vi "HFRR ADV v037.vi"() -> ()   [LabVIEW 2025] (continued)
        n1681 = VISA Close(VISA resource name=w2091, error in (no error)=w2090) -> (error out=w2093:errorcluster)
        n1682 = call <vilib>:"Clear Errors.vi"("error in (no error)"=w2093) -> ()  [unwired: 5 in, 2 out]
        n1683 = local write "Port 2a"(FALSE ("Port 2a")) -> ()
        n1684 = local read "Com Port 2"() -> (w2086:refnum<visa-resource-name>)
        "visa due" <- w2086
        n1685 = call-poly "VISA Configure Serial Port"("VISA resource name"=w2086, "timeout (10sec)"=w2097, "baud rate (9600)"=u32 250000 ("baud rate  2"), "data bits (8)"=u16 8 ("data bits  2"), "parity (0:none)"=w2096, "stop bits (10: 1 bit)"=w2098, "flow control (0:none)"=w2100) -> ("VISA resource name out"=w2101:refnum<visa-resource-name>, "error out"=w2102:errorcluster)  [unwired: 7 in]
        n1686 = flat-sequence {
          tunnel: w2101 -> [w2104]
          tunnel: w2102 -> [w2103]
          tunnel: [w2104] -> w2094
          tunnel: [w2103] -> w2087
          frame #0 {
            n1687 = Wait (ms)(milliseconds to wait=u32 50) -> ()  [unwired: 1 out]
          }
        }
        "Residual Due" <- ""
      }
    }
    "error out 9" <- w2028
    n1688 = local read "Quit"() -> (w2030:bool)
    "Error Due" <- w2035
  }
  n1689 = local write "FRICVALZ"(0.0 ("FRICVALZ")) -> ()
  n1690 = property on="RUN" class="Bool (strict)"("Visible"=TRUE) -> ()  [unwired: 2 in, 2 out]
  n1691 = while {
    tunnel: [w2119] -> _
    tunnel: [w2106] -> w54
    i -> [w2119]
    stop <- w2106 stop-if-true
    n1692 = local read "conststatus"() -> (w2110:dbl)
    n1693 = local read "Main Tab"() -> (w2108:T2)
    n1694 = local read "EDIT"() -> (w2125:bool)
    n1695 = local read "Rate"() -> (w2124:dbl)
    n1696 = case shown="True" w2125 {
      tunnel: [FALSE TRUE] -> _
      frame False {
      }
      frame True {
      }
    }
    n1697 = Equal?(x=w2108, y=T29."About" ("Main Tab")) -> (x = y?=w2117:bool)
    n1698 = Equal?(x=w2110, y=0.0) -> (x = y?=w2111:bool)
    n1699 = Divide(x=1.0, y=w2124) -> (x/y=w2120:dbl)
    "Time 2" <- w2120
    n1700 = case shown="True" w2111 {
      frame False {
      }
      frame True {
        # "C:\\WinDucom\\calibrate WO 2391.dcf"
        n1701 = local write "Lan flag"(22) -> ()
        n1702 = local write "conststatus"(10.0 ("rpm value : 2")) -> ()
        n1703 = String To Path(string="C:\\LAB-IQ\\calibrate WO 2465.dcf") -> (path=w2131:path)
        n1704 = Open/Create/Replace File "Open File"(file path (use dialog)=w2131) -> (refnum out=w2129:refnum<file>)  [unwired: 5 in, 2 out]
        n1705 = for {
          N: 23 -> [_]
          tunnel: w2129 -> [w2140]
          i -> [w2134]
          (unwired) TRUE ("line mode (F)")
          n1706 = Read from Text File "Read File"(file (use dialog)=w2140) -> (text=w2139:string)  [unwired: 3 in, 3 out]
          n1707 = Match Pattern(string=w2139, regular expression="]") -> (after substring=w2137:string)  [unwired: 1 in, 3 out]
          n1708 = String Subset(string=w2139, offset (0)=5, length (rest)=10 ("length (rest)")) -> (substring=w2132:string)
          n1709 = Fract/Exp String To Number(string=w2132) -> (number=w2133:dbl)  [unwired: 3 in, 1 out]
          n1710 = Match Pattern(string=w2137, regular expression="-") -> (before substring=w2135:string)  [unwired: 1 in, 3 out]
          n1711 = case shown="10" w2134 {
            tunnel: w2133 -> [_ _ _ _ _ _ _ _ _ _ w2147 _ _ _ _ _ _ _ _ _ _ _ _ _]
            tunnel: w2135 -> [_ _ _ _ w2143 w2144 w2145 _ _ _ _ _ _ _ _ _ _ _ _ _ w2148 w2149 w2150 _]
            frame 0 {
            }
            frame 1 {
            }
            frame 2 {
            }
            frame 3 {
            }
            frame 4 {
              n1712 = local write "Com Port 1"(w2143) -> ()
            }
            frame 5 {
              n1713 = local write "Com Port 2"(w2144) -> ()
              n1714 = local write "visa due"(w2144) -> ()
            }
            frame 6 {
              n1715 = String To Path(string=w2145) -> (path=w2146:path)
              n1716 = local write "File Path"(w2146) -> ()
              "String" <- w2145
            }
            frame 7 {
            }
            frame 8 {
            }
            frame 9 {
            }
            frame 10 {
              n1717 = local write "Language Selection"(w2147) -> ()
            }
            frame 11 {
            }
            frame 12 {
            }
            frame 13 {
            }
            frame 14 {
            }
            frame 15 {
            }
            frame 16 {
            }
            frame 17 {
            }
            frame 18 {
            }
            frame 21 {
            }
            frame 22 {
              n1718 = local write "Com Port 3"(w2148) -> ()
            }
            frame 20 {
              n1719 = local write "Camera Port :"(w2149) -> ()
            }
            frame 19 {
              n1720 = local write "C3 :"(w2150) -> ()
            }
            frame 23, Default {
            }
          }
        }
      }
    }
    n1721 = Select(t=u32 2500 ("milliseconds to wait"), s=w2117, f=u32 500 ("milliseconds to wait")) -> (s? t:f=w2115:u32)
    n1722 = Multiply(x=w2120, y=w2115) -> (x*y=w2122:dbl)
    n1723 = call "Elapsed Time2"("Time Target (s)"=w2122, "Auto Reset"=TRUE) -> ("Time has Elapsed"=w2112:bool)  [unwired: 10 in, 7 out]
    n1724 = case shown="True" w2112 {
      frame False {
      }
      frame True {
        n1725 = stacked-sequence {
          frame #0 {
            # "DATA PROCESSING"
            # "115 mV/N"
            n1726 = local read "Sample Temperature"() -> (w2153:dbl)
            n1727 = local read "RH Numeric:"() -> (→"Humidity ( %RH )":dbl)
            n1728 = local read "FRICVALZ"() -> (w2170:dbl)
            n1729 = local read "Friction"() -> (w2156:dbl)
            n1730 = call <vilib>:"Mean PtByPt.vi"("x"=w2153, "sample length"=100) -> ("mean"=w2152:dbl)  [unwired: 2 in, 1 out]
            "TEMP 2" <- w2152
            "TEMP 3" <- w2152
            n1731 = Subtract(x=w2156, y=w2170) -> (x-y=w2165:dbl)
            "FF 2" <- w2165
            "FF 4" <- w2165
            n1732 = local read "Ambient Temperature"() -> (→"AIR TEMP":dbl)
            n1733 = local read "TEMP"() -> (w2169:dbl)
            n1734 = local write "FF 3"(w2165) -> ()
            n1735 = Compound Arithmetic op=OR("FRICVALZ 4", "FRICVALZ 3", "FRICVALZ 2") -> (w2161:bool)
            n1736 = case shown="True" w2161 {
              tunnel: w2156 -> [_ w2176]
              frame False {
              }
              frame True {
                w2175 = FALSE ("FRICVALZ")
                n1737 = local write "FRICVALZ 3"(w2175) -> ()
                n1738 = local write "FRICVALZ 2"(w2175) -> ()
                n1739 = local write "FRICVALZ 4"(w2175) -> ()
                "FRICVALZ" <- w2176
              }
            }
            n1740 = Not A Number/Path/Refnum?(number/path/refnum=w2169) -> (NaN/Path/Refnum?=w2168:bool)
            n1741 = Not A Number/Path/Refnum?(number/path/refnum=w2165) -> (NaN/Path/Refnum?=w2167:bool)
            n1742 = Divide(x=w2165, y=1.96) -> (x/y=w2162:dbl)
            n1743 = Compound Arithmetic op=OR(w2168, w2167) -> (w2166:bool)
            n1744 = Not A Number/Path/Refnum?(number/path/refnum=w2162) -> (NaN/Path/Refnum?=w2163:bool)
            n1745 = case shown="True" w2166 {
              frame False {
              }
              frame True {
                n1746 = local write "TEMP"(0.0 ("TEMP")) -> ()
                n1747 = local write "FF 2"(0.0 ("FF 2")) -> ()
                n1748 = local write "reinit"(TRUE ("reinit")) -> ()
              }
            }
            n1749 = local write "TEMP"(w2152) -> ()
            n1750 = Select(t=0.0, s=w2163, f=w2162) -> (s? t:f=w2155:dbl)
            "COF 2" <- w2155
            n1751 = local write "COF 3"(w2155) -> ()
          }
        }
      }
    }
    n1752 = Wait (ms)(milliseconds to wait=u32 50) -> ()  [unwired: 1 out]
    n1753 = local read "Quit"() -> (w2106:bool)
    "Rate" <- 2500.0 ("No of Samples")
  }
  n1754 = while {
    tunnel: [w2196] -> _
    tunnel: [w2179] -> w56
    tunnel: w1 -> [_]
    i -> [w2196]
    stop <- w2179 stop-if-true
    # "C:\\LAB-IQ-NXT\\Scar View.exe"
    n1755 = local read "OK Button 16"() -> (w2186:bool)
    n1756 = local read "Main Tab"() -> (w2180:T2)
    n1757 = local read "service 3"() -> (w2181:bool)
    n1758 = local read "OPEN 6"() -> (w2183:bool)
    n1759 = local read "EDIT 2"() -> (w2185:bool)
    n1760 = flat-sequence {
      frame #0 {
        n1761 = stacked-sequence {
          frame #0 {
            n1762 = local read "EDIT"() -> (w2674:bool)
            n1763 = case shown="False" w2674 {
              tunnel: [u8 2 ("Disabled") u8 0 ("Disabled")] -> _
              frame False {
                w2676 = FALSE
                n1764 = local write "Password"("") -> ()
                n1765 = local write "x = y?"(w2676) -> ()
                n1766 = property on="Password" class="Str"("Visible"=w2676) -> ()  [unwired: 2 in, 2 out]
              }
              frame True {
                n1767 = property on="Password" class="Str"("Visible"=TRUE) -> ()  [unwired: 2 in, 2 out]
              }
            }
            "dipl pwd" <- "@143$\n" ("dipl pwd")
          }
          frame #1 {
          }
          frame #2 {
          }
          frame #3 {
          }
          frame #4 {
            n1768 = String To Byte Array(string="Password") -> (unsigned byte array=w2687:u8[])
            n1769 = Search 1D Array(1D array=w2687, element=u8 10) -> (index of element=w2685:i32)  [unwired: 1 in]
            n1770 = Index Array(array=w2687, index=w2685) -> (element=w2686:u8)
            n1771 = Equal?(x=w2686, y=10) -> (x = y?=w2682:bool)
            n1772 = case shown="True" w2682 {
              frame False {
              }
              frame True {
                # "password"
                # "password"
                n1773 = local read "Password"() -> (w2699:string)
                n1774 = String To Byte Array(string=w2699) -> (unsigned byte array=w2702:u8[])
                n1775 = String To Byte Array(string="@143$\n") -> (unsigned byte array=w2689:u8[])
                n1776 = Array Size(array=w2702) -> (size(s)=w2698:i32)
                n1777 = Array Size(array=w2689) -> (size(s)=w2694:i32)
                n1778 = for {
                  N: w2698 -> [_]
                  tunnel: w2702 -> [w2715]
                  tunnel: [w2713] -> w2703 mode=indexing
                  tunnel: w2698 -> [w2710]
                  i -> [w2711]
                  n1779 = Decrement(x=w2710) -> (x-1=w2709:i32)
                  n1780 = Index Array(array=w2715, index=w2711) -> (element=w2714:u8)
                  n1781 = Equal?(x=w2711, y=w2709) -> (x = y?=w2708:bool)
                  n1782 = Number To Decimal String(number=w2714) -> (decimal integer string=w2712:string)  [unwired: 1 in]
                  n1783 = Select(t="", s=w2708, f="\r") -> (s? t:f=w2705:string)
                  n1784 = Concatenate Strings(w2712, w2705) -> (w2713:string)
                }
                n1785 = for {
                  N: w2694 -> [_]
                  tunnel: w2689 -> [w2726]
                  tunnel: [w2724] -> w2692 mode=indexing
                  tunnel: w2694 -> [w2721]
                  i -> [w2722]
                  n1786 = Decrement(x=w2721) -> (x-1=w2720:i32)
                  n1787 = Index Array(array=w2726, index=w2722) -> (element=w2725:u8)
                  n1788 = Equal?(x=w2722, y=w2720) -> (x = y?=w2719:bool)
                  n1789 = Number To Decimal String(number=w2725) -> (decimal integer string=w2723:string)  [unwired: 1 in]
                  n1790 = Select(t="", s=w2719, f="\r") -> (s? t:f=w2716:string)
                  n1791 = Concatenate Strings(w2723, w2716) -> (w2724:string)
                }
                n1792 = local read "file path"() -> (w2688:path)
                n1793 = call <vilib>:"Read Characters From File.vi"("file path (dialog if empty)"=w2688) -> ("character string"=w2701:string)  [unwired: 5 in, 3 out]
                "string" <- w2701
                n1794 = flat-sequence {
                  tunnel: [w2704] -> _
                  frame #0 {
                    w2704 = ""
                    n1795 = local write "Password"(w2704) -> ()
                  }
                }
                n1796 = Concatenate Strings(w2692) -> (w2693:string)
                n1797 = Concatenate Strings(w2701) -> (w2700:string)
                n1798 = Concatenate Strings(w2703) -> (w2696:string)
                n1799 = Equal?(x=w2696, y=w2700) -> (x = y?=w2691:bool)
                n1800 = Equal?(x=w2696, y=w2693) -> (x = y?=w2697:bool)
                n1801 = Or(x=w2691, y=w2697) -> (x .or. y?=→"x = y?":bool)
              }
            }
          }
        }
        n1802 = local read "x = y?"() -> (w2672:bool)
        n1803 = And(x="EDIT", y=w2672) -> (x .and. y?=w2670:bool)
        n1804 = case shown="True" w2670 {
          tunnel: [u8 2 ("Disabled") u8 0 ("Disabled")] -> w2669
          tunnel: [w2876 TRUE ("Visible")] -> w2668
          frame False {
            w2876 = FALSE ("Visible")
            n1805 = local write "EDIT 2"(w2876) -> ()
          }
          frame True {
          }
        }
        n1806 = case shown="True" "SAVE" {
          frame False {
          }
          frame True {
            n1807 = stacked-sequence {
              seq-local: [w2731 _ _] -> [_ w2872 _]
              frame #0 {
                w2727 = 0.0 ("number")
                w2728 = 0.0 ("number")
                (unwired) i16 5 ("precision (6)")
                # "[CH1]    - FF\n[CH2]   - TEMPERATURE\n[CH3]    - Humidity\n[CH4]    - AIR TEMP\n[CH5]\\- Visa Uno\n[CH6] \\- Visa Due\n[CH7]  \\- file path\n[CH8]   - Displacement Gain\n[CHA]   - Stroke Gain\n[CHB]   - Stroke PID Gain\n[CHC]   -Language Selection\n[CHD]   -Power +\n[CHE]   -Power_\n[CHF]   -Heater\n[CHG]   -Humidity Wet\n[CHH]   -Humidity Dry\n[CHI]   -Integral Time"
                n1808 = local read "Language Selection"() -> (w2774:enum16{"English", "Russian"})
                n1809 = Path To String(path="File Path") -> (string=w2790:string)
                n1810 = Number To Fractional String(number=w2727, width (-)=i16 10 ("precision (6)"), precision (6)=i16 5) -> (F-format string=w2781:string)  [unwired: 1 in]
                n1811 = Number To Fractional String(number=w2774, width (-)=i16 10 ("precision (6)"), precision (6)=i16 5) -> (F-format string=w2770:string)  [unwired: 1 in]
                n1812 = Number To Fractional String(number=w2728, width (-)=i16 10 ("precision (6)"), precision (6)=i16 5) -> (F-format string=w2764:string)  [unwired: 1 in]
                n1813 = Number To Fractional String(number=w2728, width (-)=i16 10 ("precision (6)"), precision (6)=i16 5) -> (F-format string=w2761:string)  [unwired: 1 in]
                n1814 = Number To Fractional String(number=w2728, width (-)=i16 10 ("precision (6)"), precision (6)=i16 5) -> (F-format string=w2756:string)  [unwired: 1 in]
                n1815 = Number To Fractional String(number=w2728, width (-)=i16 10 ("precision (6)"), precision (6)=i16 5) -> (F-format string=w2753:string)  [unwired: 1 in]
                n1816 = Number To Fractional String(number=w2728, width (-)=i16 10 ("precision (6)"), precision (6)=i16 5) -> (F-format string=w2748:string)  [unwired: 1 in]
                n1817 = local read "Com Port 1"() -> (w2730:refnum<visa-resource-name>)
                n1818 = local read "Com Port 2"() -> (w2729:refnum<visa-resource-name>)
                n1819 = Concatenate Strings(w2790, "\\" ("string")) -> (w2789:string)
                n1820 = Number To Fractional String(number=w2727, width (-)=i16 10 ("precision (6)"), precision (6)=i16 5) -> (F-format string=w2822:string)  [unwired: 1 in]
                n1821 = Number To Fractional String(number=w2727, width (-)=i16 10 ("precision (6)"), precision (6)=i16 5) -> (F-format string=w2821:string)  [unwired: 1 in]
                n1822 = Number To Fractional String(number=w2727, width (-)=i16 10 ("precision (6)"), precision (6)=i16 5) -> (F-format string=w2815:string)  [unwired: 1 in]
                n1823 = Number To Fractional String(number=w2727, width (-)=i16 10 ("precision (6)"), precision (6)=i16 5) -> (F-format string=w2809:string)  [unwired: 1 in]
                n1824 = Number To Fractional String(number=w2727, width (-)=i16 10 ("precision (6)"), precision (6)=i16 5) -> (F-format string=w2782:string)  [unwired: 1 in]
                n1825 = Concatenate Strings("[CHA]" ("string"), w2781, "- Stroke Gain" ("string"), "\r") -> (w2775:string)
                n1826 = Concatenate Strings("[CHC]" ("string"), w2770, "-Language Selection" ("string"), "\r") -> (w2767:string)
                n1827 = Concatenate Strings("[CHD]" ("string"), w2764, "-Power +" ("string"), "\r") -> (w2746:string)
                n1828 = Concatenate Strings("[CHG]" ("string"), w2753, "-Humidity Wet" ("string"), "\r") -> (w2743:string)
                n1829 = Concatenate Strings("[CHH]" ("string"), w2748, "-Humidity Dry" ("string"), "\r") -> (w2742:string)
                n1830 = Concatenate Strings("[CH1]" ("string"), w2822, " - FF" ("string"), "\r") -> (w2820:string)
                n1831 = Concatenate Strings("[CH2]" ("string"), w2821, " - TEMPERATURE" ("string"), "\r") -> (w2819:string)
                n1832 = Concatenate Strings("[CH3]" ("string"), w2815, " - Humidity" ("string"), "\r") -> (w2812:string)
                n1833 = Concatenate Strings("[CH4]" ("string"), w2809, " - AIR TEMP" ("string"), "\r") -> (w2805:string)
                n1834 = Concatenate Strings("[CH5]" ("string"), w2730, "- Visa Uno" ("string"), "\r") -> (w2798:string)
                n1835 = Concatenate Strings("[CH6]" ("string"), w2729, "- Visa Due" ("string"), "\r") -> (w2793:string)
                n1836 = Concatenate Strings("[CH7]" ("string"), w2789, "- file path" ("string"), "\r") -> (w2792:string)
                n1837 = Concatenate Strings("[CH8]" ("string"), w2782, "- Displacement Gain" ("string"), "\r") -> (w2785:string)
                n1838 = Concatenate Strings("[CHE]" ("string"), w2761, "-Power_" ("string"), "\r") -> (w2745:string)
                n1839 = Concatenate Strings("[CHF]" ("string"), w2756, "-Heater" ("string"), "\r") -> (w2744:string)
                n1840 = Concatenate Strings(w2820, w2819, w2812, w2805, w2798, w2793, w2792, w2785, w2775, w2767, w2746, w2745, w2744, w2743, w2742) -> (w2731:string)
                "gain" <- w2731
              }
              frame #1 {
                w2833 = 0.0 ("number")
                n1841 = local read "Camera Port :"() -> (w2836:string)
                n1842 = local read "C3 :"() -> (w2844:refnum<visa-resource-name>)
                n1843 = local read "Com Port 3"() -> (w2845:refnum<visa-resource-name>)
                n1844 = Concatenate Strings("[CH8]" ("string"), w2836, "- Visa Camera" ("string"), "\r") -> (w2835:string)
                n1845 = Concatenate Strings("[CH7]" ("string"), w2844, "- Visa Humidity" ("string"), "\r") -> (w2840:string)
                n1846 = Number To Fractional String(number=w2833, width (-)=i16 10 ("precision (6)"), precision (6)=i16 5) -> (F-format string=w2860:string)  [unwired: 1 in]
                n1847 = Concatenate Strings("[CHL]" ("string"), w2845, "- Visa humid" ("string"), "\r") -> (w2848:string)
                n1848 = Number To Fractional String(number=w2833, width (-)=i16 10 ("precision (6)"), precision (6)=i16 5) -> (F-format string=w2867:string)  [unwired: 1 in]
                n1849 = Concatenate Strings("[CHK]" ("string"), w2860, "-TEMP INTERCEPT" ("string"), "\r") -> (w2856:string)
                n1850 = Concatenate Strings("[SNO]" ("string"), "" ("string"), "-" ("string"), "\r") -> (w2853:string)
                n1851 = Concatenate Strings("[CHJ]" ("string"), w2867, "-AIR TEMP INTERCEPT" ("string"), "\r") -> (w2857:string)
                n1852 = String To Path(string="C:\\LAB-IQ\\calibrate WO 2465.dcf") -> (path=w2846:path)
                n1853 = Concatenate Strings(w2872, w2857, w2856, w2853, w2848, w2840, w2835) -> (w2871:string)
                n1854 = call <vilib>:"Write Characters To File.vi"("append to file? (new file:F)"=FALSE, "character string"=w2871, "file path (dialog if empty)"=w2846) -> ()  [unwired: 2 in, 1 out]
              }
              frame #2 {
                n1855 = local write "Lan flag"(0.0 ("Lan flag")) -> ()
                n1856 = local write "conststatus"(0.0 ("rpm value : 2")) -> ()
                n1857 = local write "SAVE"(FALSE ("OK Button 14")) -> ()
              }
            }
          }
        }
        n1858 = property on="EDIT 2" class="Bool (strict)"("Visible"=w2668) -> ()  [unwired: 2 in, 2 out]
        n1859 = property on="SAVE" class="Bool (strict)"("Visible"=w2668) -> ()  [unwired: 2 in, 2 out]
        n1860 = property on="visa due" class="CmbBox"("Disabled"=w2669) -> ()  [unwired: 2 in, 2 out]
        n1861 = property on="File Path" class="Path"("Disabled"=w2669) -> ()  [unwired: 2 in, 2 out]
        n1862 = property on="Language Selection" class="Enum (strict)"("Visible"=w2668) -> ()  [unwired: 2 in, 2 out]
        n1863 = property on="SPEED OUT:" class="DigNum (strict)"("Disabled"=w2669) -> ()  [unwired: 2 in, 2 out]
      }
    }
    n1864 = local read "RUN"() -> (w2195:bool)
    n1865 = local read "RUN"() -> (w2193:bool)
    n1866 = case shown="True" "EDIT 3" {
      frame False {
      }
      frame True {
        n1867 = local write "EDIT 3"(FALSE ("EDIT 3")) -> ()
        n1868 = local write "Main Tab"(T2."About" ("Main Tab")) -> ()
      }
    }
    n1869 = case shown="False" w2195 {
      frame False {
        n1870 = local read "stopT"() -> (w2883:bool)
        n1871 = case shown="True" w2883 {
          frame False {
          }
          frame True {
            n1872 = local write "stopT"(FALSE) -> ()
          }
        }
      }
      frame True {
        "stopT" <- TRUE
      }
    }
    n1873 = case shown="False" w2193 {
      frame False {
      }
      frame True {
      }
    }
    n1874 = case shown="True" w2185 {
      frame False {
        n1875 = property on="Password 2" class="Str"("Visible"=FALSE) -> ()  [unwired: 2 in, 2 out]
        n1876 = local write "Password 2"("" ("Password")) -> ()
      }
      frame True {
        n1877 = property on="Password 2" class="Str"("Visible"=TRUE) -> ()  [unwired: 2 in, 2 out]
        n1878 = Equal?(x="Password 2", y="HFRR1234") -> (x = y?=w2208:bool)
        n1879 = case shown="True" w2208 {
          tunnel: "Password 2" -> [w2211 _]
          frame False {
            n1880 = String Length(string=w2211) -> (length=w2212:i32)
            n1881 = Greater Than 0?(x=w2212) -> (x > 0?=w2210:bool)
            n1882 = case shown="False" w2210 {
              frame False {
                n1883 = property on="Password 2" class="Str"("Caption.Text"="Password (Advance Setting)") -> ()  [unwired: 2 in, 2 out]
              }
              frame True {
                n1884 = property on="Password 2" class="Str"("Caption.Text"="Incorrect Password!") -> ()  [unwired: 2 in, 2 out]
              }
            }
          }
          frame True {
            n1885 = local write "EDIT 2"(FALSE ("EDIT 2")) -> ()
            n1886 = local write "Password 2"("" ("Password")) -> ()
            n1887 = local write "Main Tab"(T2."Advance" ("Main Tab")) -> ()
            n1888 = local write "Main Dashboard Buttons"(T1."Advance" ("Main Dashboard Buttons")) -> ()
          }
        }
      }
    }
    n1889 = case shown="True" "Prog Uno" {
      frame False {
      }
      frame True {
        n1890 = stacked-sequence {
          frame #0 {
            n1891 = Delete(path (use dialog)=path "C:/LAB-IQ-NXT/UNOCOMPILE.bat" ("working directory")) -> ()  [unwired: 4 in, 3 out]
          }
          frame #1 {
            n1892 = local read "Com Port 1"() -> (w2650:refnum<visa-resource-name>)
            n1893 = Concatenate Strings("cmd.exe /c \"mode " ("command line"), w2650, ":1200,n,8,1\"\n" ("command line")) -> (w2655:string)
            n1894 = Concatenate Strings(w2655, "CD\\\nCD WinDucom\navrdude -C avrdude.conf -v -patmega328p -carduino -P" ("command line"), w2650, " -b115200 -D -Uflash:w:UNO_V20.hex:i\n" ("command line"), "\r") -> (w2657:string)
            "STR" <- w2657
            n1895 = call <vilib>:"Write Characters To File.vi"("append to file? (new file:F)"=FALSE, "character string"=w2657, "file path (dialog if empty)"=path "C:/LAB-IQ/UNOCOMPILE.bat" ("working directory")) -> ()  [unwired: 2 in, 1 out]
          }
          frame #2 {
            n1896 = disable-structure shown="Disabled" {
              frame Disabled {
                w2661 = "cmd.exe  /c \"C:\\LAB-IQ-NXT\\UNOCOMPILE.bat\"" ("string")
                n1897 = local write "Prog Uno"(FALSE ("run minimized? (F)")) -> ()
                n1898 = call <vilib>:"System Exec.vi"("expected output size  (4096)"=u32 65535, "run minimized? (F)"=FALSE, "wait until completion? (T)"=TRUE ("run minimized? (F)"), "working directory"=path "C:/LAB-IQ-NXT", "standard input"=w2661, "command line"=w2661) -> ("error out"=w2660:errorcluster, "standard output"=→"String 42":string)  [unwired: 2 in, 2 out]
                "error out 3" <- w2660
                n1899 = flat-sequence {
                  tunnel: w2660 -> [_]
                  frame #0 {
                  }
                }
              }
              frame Enabled {
              }
            }
          }
        }
      }
    }
    n1900 = case shown="\"ISO 12156\"" "TEST STANDARD" {
      frame "ASTM D6079", Default {
        w2630 = 50.0 ("Hz")
        w2631 = 53.0 ("Set Rh")
        w2633 = 1.0 ("Set Strk")
        w2632 = 60.0 ("Set Temp")
        # "astm hide"
        n1901 = local write "NORMAL LOAD"(200.0 ("NORMAL LOAD")) -> ()
        n1902 = local write "Set Strk"(w2633) -> ()
        n1903 = local write "Set Hz"(w2630) -> ()
        n1904 = local write "Set Temp"(w2632) -> ()
        n1905 = local write "Set Rh"(w2631) -> ()
        n1906 = local write "test time"(75.0 ("test time")) -> ()
        n1907 = local write "Set Stroke:"(w2633) -> ()
        n1908 = local write "Set Humidity:"(w2631) -> ()
        n1909 = local write "Set Frequency:"(w2630) -> ()
        n1910 = local write "Set Temperature:"(w2632) -> ()
        "Test Standard" <- "ASTM D6079" ("Test Standard 2")
      }
      frame "ISO 12156" {
        n1911 = local write "Set Strk"(1.0 ("Set Strk")) -> ()
        n1912 = local write "NORMAL LOAD"(200.0 ("NORMAL LOAD")) -> ()
        n1913 = local write "Set Temp"(60.0 ("Set Temp")) -> ()
        n1914 = local write "test time"(75.0 ("test time")) -> ()
        n1915 = local write "Set Hz"(50.0 ("Hz")) -> ()
        n1916 = local write "Set Rh"(53.0 ("Set Rh")) -> ()
      }
      frame "CEC F-096-A-06" {
        n1917 = local write "Set Strk"(1.0 ("Set Strk")) -> ()
        n1918 = local write "NORMAL LOAD"(200.0 ("NORMAL LOAD")) -> ()
        n1919 = local write "Set Temp"(60.0 ("Set Temp")) -> ()
        n1920 = local write "test time"(75.0 ("test time")) -> ()
        n1921 = local write "Set Hz"(50.0 ("Hz")) -> ()
        n1922 = local write "Set Rh"(53.0 ("Set Rh")) -> ()
      }
      frame "Custom" {
      }
    }
    n1923 = Or(x=w2183, y=w2181) -> (x .or. y?=w2182:bool)
    n1924 = case shown="\"About\"" w2180 {
      tunnel: [T29."Acquire" ("Main Tab") T29."Compare Files" ("Main Tab") T29."About" ("Main Tab")] -> w2191
      frame "Acquire", Default {
      }
      frame "Compare Files" {
      }
      frame "About" {
      }
    }
    n1925 = Or(x=w2186, y="OPEN") -> (x .or. y?=w2187:bool)
    n1926 = case shown="True" w2187 {
      tunnel: w2186 -> [_ w2219]
      frame False {
      }
      frame True {
        n1927 = stacked-sequence {
          tunnel: w2219 -> [_ w2286 _ _]
          frame #0 {
            w2235 = "  " ("String 6")
            n1928 = local write "OPEN"(FALSE ("open")) -> ()
            n1929 = local read "string1 2"() -> (w2223:string)
            n1930 = local read "string1 3"() -> (w2222:string)
            n1931 = local read "string1 4"() -> (w2221:string)
            n1932 = property on="OPEN" class="Bool (strict)"("Visible"=FALSE) -> ()  [unwired: 2 in, 2 out]
            n1933 = local write "String 6"(w2235) -> ()
            n1934 = local write "String 7"(w2235) -> ()
            n1935 = local write "String 8"(w2235) -> ()
            n1936 = local write "String 12"(w2235) -> ()
            n1937 = local read "OK Button 16"() -> (w2220:bool)
            n1938 = String To Path(string=w2223) -> (path=w2231:path)
            n1939 = String To Path(string=w2222) -> (path=w2230:path)
            n1940 = String To Path(string=w2221) -> (path=w2229:path)
            n1941 = case shown="True" w2220 {
              tunnel: [w2236 w2237] -> w2224
              frame False {
                n1942 = local read "string1"() -> (w2236:string)
              }
              frame True {
                n1943 = local read "String Indicator 4"() -> (w2237:string)
              }
            }
            n1944 = Open/Create/Replace File "Open File"(file path (use dialog)=w2231) -> (refnum out=w2227:refnum<file>)  [unwired: 5 in, 2 out]
            n1945 = Open/Create/Replace File "Open File"(file path (use dialog)=w2230) -> (refnum out=w2226:refnum<file>)  [unwired: 5 in, 2 out]
            n1946 = Open/Create/Replace File "Open File"(file path (use dialog)=w2229) -> (refnum out=w2225:refnum<file>)  [unwired: 5 in, 2 out]
            n1947 = while {
              tunnel: w2227 -> [w2249]
              i -> [w2245]
              stop <- w2244 continue-if-true
              (unwired) TRUE ("line mode (F)")
              n1948 = Read from Text File "Read File"(file (use dialog)=w2249) -> (text=w2246:string)  [unwired: 3 in, 3 out]
              n1949 = local write "Numeric 11"(w2245) -> ()
              n1950 = String Length(string=w2246) -> (length=w2248:i32)
              n1951 = Greater?(x=w2248, y=1) -> (0:w2244:bool)
            }
            n1952 = while {
              tunnel: w2226 -> [w2255]
              i -> [w2251]
              stop <- w2250 continue-if-true
              (unwired) TRUE ("line mode (F)")
              n1953 = Read from Text File "Read File"(file (use dialog)=w2255) -> (text=w2252:string)  [unwired: 3 in, 3 out]
              n1954 = local write "Numeric 12"(w2251) -> ()
              n1955 = String Length(string=w2252) -> (length=w2254:i32)
              n1956 = Greater?(x=w2254, y=1) -> (0:w2250:bool)
            }
            n1957 = while {
              tunnel: w2225 -> [w2261]
              i -> [w2257]
              stop <- w2256 continue-if-true
              (unwired) TRUE ("line mode (F)")
              n1958 = Read from Text File "Read File"(file (use dialog)=w2261) -> (text=w2258:string)  [unwired: 3 in, 3 out]
              n1959 = local write "Numeric 13"(w2257) -> ()
              n1960 = String Length(string=w2258) -> (length=w2260:i32)
              n1961 = Greater?(x=w2260, y=1) -> (0:w2256:bool)
            }
            n1962 = String To Path(string=w2224) -> (path=w2232:path)
            n1963 = Open/Create/Replace File "Open File"(file path (use dialog)=w2232) -> (refnum out=w2228:refnum<file>)  [unwired: 5 in, 2 out]
            n1964 = while {
              tunnel: w2228 -> [w2243]
              i -> [w2239]
              stop <- w2238 continue-if-true
              (unwired) TRUE ("line mode (F)")
              n1965 = Read from Text File "Read File"(file (use dialog)=w2243) -> (text=w2240:string)  [unwired: 3 in, 3 out]
              n1966 = local write "Numeric 8"(w2239) -> ()
              n1967 = String Length(string=w2240) -> (length=w2242:i32)
              n1968 = Greater?(x=w2242, y=1) -> (0:w2238:bool)
            }
          }
          frame #1 {
            w2413 = FALSE ("ACTUAL   MERGE")
            # "Sample Temp"
            # "ECR"
            # "COF"
            # "Time\nCOF\nFF\nTemp"
            n1969 = case shown="True" w2286 {
              tunnel: [w2433 w2434] -> w2287
              frame False {
                n1970 = local read "string1"() -> (w2433:string)
              }
              frame True {
                n1971 = local read "String Indicator 4"() -> (w2434:string)
              }
            }
            n1972 = local read "string1 3"() -> (w2331:string)
            n1973 = String To Path(string=w2287) -> (path=w2418:path)
            n1974 = String To Path(string=w2331) -> (path=w2429:path)
            n1975 = local read "Numeric 12"() -> (w2415:i32)
            n1976 = local read "Numeric 8"() -> (w2417:i32)
            n1977 = local read "string1 2"() -> (w2332:string)
            n1978 = local read "string1 4"() -> (w2330:string)
            n1979 = Open/Create/Replace File "Open File"(file path (use dialog)=w2418) -> (refnum out=w2432:refnum<file>, error out=w2431:errorcluster)  [unwired: 5 in, 1 out]
            n1980 = Open/Create/Replace File "Open File"(file path (use dialog)=w2429) -> (refnum out=w2425:refnum<file>, error out=w2426:errorcluster)  [unwired: 5 in, 1 out]
            n1981 = for {
              N: w2417 -> [_]
              tunnel: w2432 -> [w2580]
              tunnel: w2431 -> [w2579]
              tunnel: [w2569] -> w2344 mode=indexing
              tunnel: [w2567] -> w2401 mode=indexing
              tunnel: [w2568] -> w2396 mode=indexing
              tunnel: w2413 -> [_]
              tunnel: [w2561] -> w2398 mode=indexing
              tunnel: [w2557] -> w2367 mode=indexing
              tunnel: [w2553] -> w2342 mode=indexing
              tunnel: [w2549] -> w2323 mode=indexing
              tunnel: [w2544] -> w2283 mode=indexing
              (unwired) TRUE ("line mode (F)")
              # "freq"
              # "Stroke"
              # "Time"
              # "CoF"
              # "Humidity"
              # "Temp"
              # "Air Temp"
              # "ECR"
              n1982 = Read from Text File "Read File"(file (use dialog)=w2580, error in=w2579) -> (text=w2545:string)  [unwired: 2 in, 3 out]
              n1983 = local write "String 6"(w2545) -> ()
              n1984 = String Subset(string=w2545, offset (0)=0, length (rest)=14 ("length (rest)")) -> (substring=w2573:string)
              n1985 = String Subset(string=w2545, offset (0)=35, length (rest)=9 ("length (rest)")) -> (substring=w2570:string)
              n1986 = String Subset(string=w2545, offset (0)=15, length (rest)=9 ("length (rest)")) -> (substring=w2576:string)
              n1987 = Fract/Exp String To Number(string=w2573) -> (number=w2569:dbl)  [unwired: 3 in, 1 out]
              n1988 = Fract/Exp String To Number(string=w2570) -> (number=w2568:dbl)  [unwired: 3 in, 1 out]
              n1989 = Fract/Exp String To Number(string=w2576) -> (number=w2567:dbl)  [unwired: 3 in, 1 out]
              n1990 = String Subset(string=w2545, offset (0)=85, length (rest)=9 ("length (rest)")) -> (substring=w2546:string)
              n1991 = String Subset(string=w2545, offset (0)=25, length (rest)=9 ("length (rest)")) -> (substring=w2552:string)
              n1992 = String Subset(string=w2545, offset (0)=55, length (rest)=9 ("length (rest)")) -> (substring=w2554:string)
              n1993 = String Subset(string=w2545, offset (0)=45, length (rest)=9 ("length (rest)")) -> (substring=w2560:string)
              n1994 = String Subset(string=w2545, offset (0)=65, length (rest)=9 ("length (rest)")) -> (substring=w2566:string)
              n1995 = Fract/Exp String To Number(string=w2552) -> (number=w2549:dbl)  [unwired: 3 in, 1 out]
              n1996 = Fract/Exp String To Number(string=w2546) -> (number=w2544:dbl)  [unwired: 3 in, 1 out]
              n1997 = Fract/Exp String To Number(string=w2554) -> (number=w2553:dbl)  [unwired: 3 in, 1 out]
              n1998 = Fract/Exp String To Number(string=w2560) -> (number=w2557:dbl)  [unwired: 3 in, 1 out]
              n1999 = Fract/Exp String To Number(string=w2566) -> (number=w2563:dbl)  [unwired: 3 in, 1 out]
              n2000 = Add(x=w2563, y=0.0) -> (x+y=w2561:dbl)
            }
            n2001 = for {
              N: w2415 -> [_]
              tunnel: w2426 -> [w2506]
              tunnel: w2425 -> [w2505]
              tunnel: [w2495] -> w2384 mode=indexing
              tunnel: [w2493] -> w2382 mode=indexing
              tunnel: [w2494] -> w2378 mode=indexing
              tunnel: w2413 -> [_]
              tunnel: [w2487] -> w2380 mode=indexing
              tunnel: [w2483] -> w2362 mode=indexing
              tunnel: [w2479] -> w2338 mode=indexing
              tunnel: [w2476] -> w2319 mode=indexing
              tunnel: [w2472] -> w2278 mode=indexing
              (unwired) 9 ("length (rest)")
              (unwired) 9 ("length (rest)")
              (unwired) TRUE ("line mode (F)")
              n2002 = Read from Text File "Read File"(file (use dialog)=w2505, error in=w2506) -> (text=w2473:string)  [unwired: 2 in, 3 out]
              n2003 = local write "String 8"(w2473) -> ()
              n2004 = String Subset(string=w2473, offset (0)=85) -> (substring=w2475:string)  [unwired: 1 in]
              n2005 = String Subset(string=w2473, offset (0)=35, length (rest)=9 ("length (rest)")) -> (substring=w2496:string)
              n2006 = String Subset(string=w2473, offset (0)=55, length (rest)=9 ("length (rest)")) -> (substring=w2481:string)
              n2007 = String Subset(string=w2473, offset (0)=25) -> (substring=w2477:string)  [unwired: 1 in]
              n2008 = String Subset(string=w2473, offset (0)=15, length (rest)=9 ("length (rest)")) -> (substring=w2502:string)
              n2009 = String Subset(string=w2473, offset (0)=0, length (rest)=14 ("length (rest)")) -> (substring=w2499:string)
              n2010 = String Subset(string=w2473, offset (0)=45, length (rest)=9 ("length (rest)")) -> (substring=w2486:string)
              n2011 = String Subset(string=w2473, offset (0)=65, length (rest)=9 ("length (rest)")) -> (substring=w2492:string)
              n2012 = Fract/Exp String To Number(string=w2475) -> (number=w2472:dbl)  [unwired: 3 in, 1 out]
              n2013 = Fract/Exp String To Number(string=w2496) -> (number=w2494:dbl)  [unwired: 3 in, 1 out]
              n2014 = Fract/Exp String To Number(string=w2481) -> (number=w2479:dbl)  [unwired: 3 in, 1 out]
              n2015 = Fract/Exp String To Number(string=w2477) -> (number=w2476:dbl)  [unwired: 3 in, 1 out]
              n2016 = Fract/Exp String To Number(string=w2502) -> (number=w2493:dbl)  [unwired: 3 in, 1 out]
              n2017 = Fract/Exp String To Number(string=w2499) -> (number=w2495:dbl)  [unwired: 3 in, 1 out]
              n2018 = Fract/Exp String To Number(string=w2486) -> (number=w2483:dbl)  [unwired: 3 in, 1 out]
              n2019 = Fract/Exp String To Number(string=w2492) -> (number=w2489:dbl)  [unwired: 3 in, 1 out]
              n2020 = Add(x=w2489, y=0.0) -> (x+y=w2487:dbl)
            }
            n2021 = String To Path(string=w2332) -> (path=w2430:path)
            n2022 = String To Path(string=w2330) -> (path=w2424:path)
            n2023 = local read "Numeric 11"() -> (w2414:i32)
            n2024 = local read "Numeric 13"() -> (w2416:i32)
            n2025 = Open/Create/Replace File "Open File"(file path (use dialog)=w2430) -> (refnum out=w2428:refnum<file>, error out=w2427:errorcluster)  [unwired: 5 in, 1 out]
            n2026 = Open/Create/Replace File "Open File"(file path (use dialog)=w2424) -> (refnum out=w2423:refnum<file>, error out=w2422:errorcluster)  [unwired: 5 in, 1 out]
            n2027 = for {
              N: w2414 -> [_]
              tunnel: w2428 -> [w2543]
              tunnel: w2427 -> [w2542]
              tunnel: [w2532] -> w2394 mode=indexing
              tunnel: [w2530] -> w2392 mode=indexing
              tunnel: [w2531] -> w2387 mode=indexing
              tunnel: w2413 -> [_]
              tunnel: [w2524] -> w2389 mode=indexing
              tunnel: [w2520] -> w2365 mode=indexing
              tunnel: [w2516] -> w2340 mode=indexing
              tunnel: [w2512] -> w2321 mode=indexing
              tunnel: [w2507] -> w2279 mode=indexing
              (unwired) TRUE ("line mode (F)")
              n2028 = Read from Text File "Read File"(file (use dialog)=w2543, error in=w2542) -> (text=w2508:string)  [unwired: 2 in, 3 out]
              n2029 = local write "String 7"(w2508) -> ()
              n2030 = String Subset(string=w2508, offset (0)=85, length (rest)=9 ("length (rest)")) -> (substring=w2511:string)
              n2031 = String Subset(string=w2508, offset (0)=35, length (rest)=9 ("length (rest)")) -> (substring=w2533:string)
              n2032 = String Subset(string=w2508, offset (0)=55, length (rest)=9 ("length (rest)")) -> (substring=w2519:string)
              n2033 = String Subset(string=w2508, offset (0)=25, length (rest)=9 ("length (rest)")) -> (substring=w2513:string)
              n2034 = String Subset(string=w2508, offset (0)=45, length (rest)=9 ("length (rest)")) -> (substring=w2521:string)
              n2035 = String Subset(string=w2508, offset (0)=0, length (rest)=14 ("length (rest)")) -> (substring=w2536:string)
              n2036 = String Subset(string=w2508, offset (0)=15, length (rest)=9 ("length (rest)")) -> (substring=w2539:string)
              n2037 = String Subset(string=w2508, offset (0)=65, length (rest)=9 ("length (rest)")) -> (substring=w2525:string)
              n2038 = Fract/Exp String To Number(string=w2511) -> (number=w2507:dbl)  [unwired: 3 in, 1 out]
              n2039 = Fract/Exp String To Number(string=w2533) -> (number=w2531:dbl)  [unwired: 3 in, 1 out]
              n2040 = Fract/Exp String To Number(string=w2519) -> (number=w2516:dbl)  [unwired: 3 in, 1 out]
              n2041 = Fract/Exp String To Number(string=w2513) -> (number=w2512:dbl)  [unwired: 3 in, 1 out]
              n2042 = Fract/Exp String To Number(string=w2521) -> (number=w2520:dbl)  [unwired: 3 in, 1 out]
              n2043 = Fract/Exp String To Number(string=w2536) -> (number=w2532:dbl)  [unwired: 3 in, 1 out]
              n2044 = Fract/Exp String To Number(string=w2539) -> (number=w2530:dbl)  [unwired: 3 in, 1 out]
              n2045 = Fract/Exp String To Number(string=w2525) -> (number=w2528:dbl)  [unwired: 3 in, 1 out]
              n2046 = Add(x=w2528, y=0.0) -> (x+y=w2524:dbl)
            }
            n2047 = for {
              N: w2416 -> [_]
              tunnel: w2423 -> [w2471]
              tunnel: w2422 -> [w2470]
              tunnel: [w2460] -> w2376 mode=indexing
              tunnel: [w2459] -> w2369 mode=indexing
              tunnel: w2413 -> [_]
              tunnel: [w2448] -> w2374 mode=indexing
              tunnel: [w2453] -> w2371 mode=indexing
              tunnel: [w2449] -> w2361 mode=indexing
              tunnel: [w2444] -> w2336 mode=indexing
              tunnel: [w2440] -> w2317 mode=indexing
              tunnel: [w2435] -> w2277 mode=indexing
              (unwired) 1.0 ("x")
              (unwired) TRUE ("line mode (F)")
              n2048 = Read from Text File "Read File"(file (use dialog)=w2471, error in=w2470) -> (text=w2436:string)  [unwired: 2 in, 3 out]
              n2049 = local write "String 12"(w2436) -> ()
              n2050 = String Subset(string=w2436, offset (0)=85, length (rest)=9 ("length (rest)")) -> (substring=w2438:string)
              n2051 = String Subset(string=w2436, offset (0)=35, length (rest)=9 ("length (rest)")) -> (substring=w2461:string)
              n2052 = String Subset(string=w2436, offset (0)=55, length (rest)=9 ("length (rest)")) -> (substring=w2446:string)
              n2053 = String Subset(string=w2436, offset (0)=25, length (rest)=9 ("length (rest)")) -> (substring=w2442:string)
              n2054 = String Subset(string=w2436, offset (0)=45, length (rest)=9 ("length (rest)")) -> (substring=w2451:string)
              n2055 = String Subset(string=w2436, offset (0)=15, length (rest)=9 ("length (rest)")) -> (substring=w2467:string)
              n2056 = String Subset(string=w2436, offset (0)=0, length (rest)=14 ("length (rest)")) -> (substring=w2464:string)
              n2057 = String Subset(string=w2436, offset (0)=65, length (rest)=9 ("length (rest)")) -> (substring=w2454:string)
              n2058 = Fract/Exp String To Number(string=w2438) -> (number=w2435:dbl)  [unwired: 3 in, 1 out]
              n2059 = Fract/Exp String To Number(string=w2461) -> (number=w2459:dbl)  [unwired: 3 in, 1 out]
              n2060 = Fract/Exp String To Number(string=w2446) -> (number=w2444:dbl)  [unwired: 3 in, 1 out]
              n2061 = Fract/Exp String To Number(string=w2442) -> (number=w2440:dbl)  [unwired: 3 in, 1 out]
              n2062 = Fract/Exp String To Number(string=w2451) -> (number=w2449:dbl)  [unwired: 3 in, 1 out]
              n2063 = Fract/Exp String To Number(string=w2467) -> (number=w2448:dbl)  [unwired: 3 in, 1 out]
              n2064 = Fract/Exp String To Number(string=w2464) -> (number=w2460:dbl)  [unwired: 3 in, 1 out]
              n2065 = Fract/Exp String To Number(string=w2454) -> (number=w2457:dbl)  [unwired: 3 in, 1 out]
              n2066 = Add(x=w2457, y=0.0) -> (x+y=w2453:dbl)
            }
            n2067 = Delete From Array(array=w2319, index=0) -> (array with subset deleted=w2292:dbl[])  [unwired: 1 in, 1 out]
            n2068 = Delete From Array(array=w2382, index=0) -> (array with subset deleted=w2355:dbl[])  [unwired: 1 in, 1 out]
            n2069 = Delete From Array(array=w2362, index=0) -> (array with subset deleted=w2350:dbl[])  [unwired: 1 in, 1 out]
            n2070 = Delete From Array(array=w2380, index=0) -> (array with subset deleted=w2381:dbl[])  [unwired: 1 in, 1 out]
            n2071 = call-poly <vilib>:"Mean.vi"("X"=w2292) -> ("mean"=→"КОФ2 4":dbl)  [unwired: 1 out]
            n2072 = call-poly <vilib>:"Mean.vi"("X"=w2355) -> ("mean"=→"КОФ3":dbl)  [unwired: 1 out]
            n2073 = call-poly <vilib>:"Mean.vi"("X"=w2350) -> ("mean"=→"CP3":dbl)  [unwired: 1 out]
            n2074 = Delete From Array(array=w2344, index=0) -> (array with subset deleted=w2271:dbl[])  [unwired: 1 in, 1 out]
            n2075 = Delete From Array(array=w2283, index=0) -> (array with subset deleted=w2270:dbl[])  [unwired: 1 in, 1 out]
            n2076 = Delete From Array(array=w2323, index=0) -> (array with subset deleted=w2294:dbl[])  [unwired: 1 in, 1 out]
            n2077 = Delete From Array(array=w2401, index=0) -> (array with subset deleted=w2356:dbl[])  [unwired: 1 in, 1 out]
            n2078 = Delete From Array(array=w2367, index=0) -> (array with subset deleted=w2352:dbl[])  [unwired: 1 in, 1 out]
            "array w/ subset deleted" <- w2352
            n2079 = Delete From Array(array=w2398, index=0) -> (array with subset deleted=w2399:dbl[])  [unwired: 1 in, 1 out]
            n2080 = call-poly <vilib>:"Mean.vi"("X"=w2294) -> ("mean"=→"КОФ2 2":dbl)  [unwired: 1 out]
            n2081 = call-poly <vilib>:"Mean.vi"("X"=w2356) -> ("mean"=→"КОФ1":dbl)  [unwired: 1 out]
            n2082 = Bundle "Bundle"(w2271, w2270) -> (w2276:cluster{dbl[], dbl[]})  [unwired: 1 in]
            n2083 = Bundle "Bundle"(w2271, w2399) -> (w2263:cluster{dbl[], dbl[]})  [unwired: 1 in]
            n2084 = Delete From Array(array=w2278, index=0) -> (array with subset deleted=w2266:dbl[])  [unwired: 1 in, 1 out]
            n2085 = Delete From Array(array=w2279, index=0) -> (array with subset deleted=w2268:dbl[])  [unwired: 1 in, 1 out]
            n2086 = Delete From Array(array=w2389, index=0) -> (array with subset deleted=w2390:dbl[])  [unwired: 1 in, 1 out]
            n2087 = Delete From Array(array=w2277, index=0) -> (array with subset deleted=w2264:dbl[])  [unwired: 1 in, 1 out]
            n2088 = Delete From Array(array=w2371, index=0) -> (array with subset deleted=w2372:dbl[])  [unwired: 1 in, 1 out]
            n2089 = Delete From Array(array=w2396, index=0) -> (array with subset deleted=w2302:dbl[])  [unwired: 1 in, 1 out]
            n2090 = Delete From Array(array=w2342, index=0) -> (array with subset deleted=w2298:dbl[])  [unwired: 1 in, 1 out]
            n2091 = Delete From Array(array=w2378, index=0) -> (array with subset deleted=w2300:dbl[])  [unwired: 1 in, 1 out]
            n2092 = Delete From Array(array=w2338, index=0) -> (array with subset deleted=w2296:dbl[])  [unwired: 1 in, 1 out]
            n2093 = Delete From Array(array=w2387, index=0) -> (array with subset deleted=w2301:dbl[])  [unwired: 1 in, 1 out]
            n2094 = Delete From Array(array=w2340, index=0) -> (array with subset deleted=w2297:dbl[])  [unwired: 1 in, 1 out]
            n2095 = Delete From Array(array=w2321, index=0) -> (array with subset deleted=w2293:dbl[])  [unwired: 1 in, 1 out]
            n2096 = Delete From Array(array=w2365, index=0) -> (array with subset deleted=w2351:dbl[])  [unwired: 1 in, 1 out]
            n2097 = Delete From Array(array=w2392, index=0) -> (array with subset deleted=w2353:dbl[])  [unwired: 1 in, 1 out]
            n2098 = Delete From Array(array=w2369, index=0) -> (array with subset deleted=w2299:dbl[])  [unwired: 1 in, 1 out]
            n2099 = Delete From Array(array=w2336, index=0) -> (array with subset deleted=w2295:dbl[])  [unwired: 1 in, 1 out]
            n2100 = Delete From Array(array=w2317, index=0) -> (array with subset deleted=w2291:dbl[])  [unwired: 1 in, 1 out]
            n2101 = Delete From Array(array=w2361, index=0) -> (array with subset deleted=w2349:dbl[])  [unwired: 1 in, 1 out]
            n2102 = Delete From Array(array=w2374, index=0) -> (array with subset deleted=w2354:dbl[])  [unwired: 1 in, 1 out]
            n2103 = Delete From Array(array=w2384, index=0) -> (array with subset deleted=w2267:dbl[])  [unwired: 1 in, 1 out]
            n2104 = Delete From Array(array=w2394, index=0) -> (array with subset deleted=w2269:dbl[])  [unwired: 1 in, 1 out]
            n2105 = Delete From Array(array=w2376, index=0) -> (array with subset deleted=w2265:dbl[])  [unwired: 1 in, 1 out]
            n2106 = Bundle "Bundle"(w2271, w2302) -> (w2289:cluster{dbl[], dbl[]})  [unwired: 1 in]
            n2107 = Bundle "Bundle"(w2271, w2356) -> (w2290:cluster{dbl[], dbl[]})  [unwired: 1 in]
            n2108 = Bundle "Bundle"(w2302, w2298) -> (w2304:cluster{dbl[], dbl[]})  [unwired: 1 in]
            n2109 = Bundle "Bundle"(w2267, w2266) -> (w2274:cluster{dbl[], dbl[]})  [unwired: 1 in]
            n2110 = Bundle "Bundle"(w2300, w2296) -> (w2306:cluster{dbl[], dbl[]})  [unwired: 1 in]
            n2111 = Bundle "Bundle"(w2267, w2300) -> (w2410:cluster{dbl[], dbl[]})  [unwired: 1 in]
            n2112 = Bundle "Bundle"(w2267, w2296) -> (w2334:cluster{dbl[], dbl[]})  [unwired: 1 in]
            n2113 = Bundle "Bundle"(w2267, w2355) -> (w2420:cluster{dbl[], dbl[]})  [unwired: 1 in]
            n2114 = Bundle "Bundle"(w2267, w2350) -> (w2358:cluster{dbl[], dbl[]})  [unwired: 1 in]
            n2115 = Bundle "Bundle"(w2267, w2381) -> (w2405:cluster{dbl[], dbl[]})  [unwired: 1 in]
            n2116 = Bundle "Bundle"(w2301, w2297) -> (w2305:cluster{dbl[], dbl[]})  [unwired: 1 in]
            n2117 = Bundle "Bundle"(w2269, w2268) -> (w2275:cluster{dbl[], dbl[]})  [unwired: 1 in]
            n2118 = Bundle "Bundle"(w2269, w2301) -> (w2412:cluster{dbl[], dbl[]})  [unwired: 1 in]
            n2119 = Bundle "Bundle"(w2269, w2297) -> (w2335:cluster{dbl[], dbl[]})  [unwired: 1 in]
            n2120 = Bundle "Bundle"(w2269, w2351) -> (w2359:cluster{dbl[], dbl[]})  [unwired: 1 in]
            n2121 = Bundle "Bundle"(w2269, w2353) -> (w2421:cluster{dbl[], dbl[]})  [unwired: 1 in]
            n2122 = Bundle "Bundle"(w2269, w2390) -> (w2403:cluster{dbl[], dbl[]})  [unwired: 1 in]
            n2123 = Bundle "Bundle"(w2299, w2295) -> (w2307:cluster{dbl[], dbl[]})  [unwired: 1 in]
            n2124 = Bundle "Bundle"(w2265, w2264) -> (w2273:cluster{dbl[], dbl[]})  [unwired: 1 in]
            n2125 = Bundle "Bundle"(w2265, w2299) -> (w2411:cluster{dbl[], dbl[]})  [unwired: 1 in]
            n2126 = Bundle "Bundle"(w2265, w2295) -> (w2333:cluster{dbl[], dbl[]})  [unwired: 1 in]
            n2127 = Bundle "Bundle"(w2265, w2349) -> (w2357:cluster{dbl[], dbl[]})  [unwired: 1 in]
            n2128 = Bundle "Bundle"(w2265, w2354) -> (w2419:cluster{dbl[], dbl[]})  [unwired: 1 in]
            n2129 = Bundle "Bundle"(w2265, w2372) -> (w2404:cluster{dbl[], dbl[]})  [unwired: 1 in]
            n2130 = call-poly <vilib>:"Mean.vi"("X"=w2352) -> ("mean"=→"CP1":dbl)  [unwired: 1 out]
            n2131 = call-poly <vilib>:"Mean.vi"("X"=w2293) -> ("mean"=→"КОФ2 3":dbl)  [unwired: 1 out]
            n2132 = call-poly <vilib>:"Mean.vi"("X"=w2351) -> ("mean"=→"CP2":dbl)  [unwired: 1 out]
            n2133 = call-poly <vilib>:"Mean.vi"("X"=w2353) -> ("mean"=→"КОФ2":dbl)  [unwired: 1 out]
            n2134 = call-poly <vilib>:"Mean.vi"("X"=w2291) -> ("mean"=→"КОФ2 5":dbl)  [unwired: 1 out]
            n2135 = call-poly <vilib>:"Mean.vi"("X"=w2349) -> ("mean"=→"CP4":dbl)  [unwired: 1 out]
            n2136 = call-poly <vilib>:"Mean.vi"("X"=w2354) -> ("mean"=→"КОФ4":dbl)  [unwired: 1 out]
            n2137 = Bundle "Bundle"(w2271, w2298) -> (w2262:cluster{dbl[], dbl[]})  [unwired: 1 in]
            n2138 = Bundle "Bundle"(w2271, w2352) -> (w2285:cluster{dbl[], dbl[]})  [unwired: 1 in]
            n2139 = Build Array "Build Array"(w2262, w2285) -> (w2288:cluster{dbl[], dbl[]}[])
            "XY Graph 17" <- w2288
            n2140 = Build Array "Build Array"(w2276, w2275, w2274, w2273) -> (→"Frequency ( Hz )":cluster{dbl[], dbl[]}[])
            n2141 = Build Array "Build Array"(w2304, w2305, w2306, w2307) -> (→"Air Temp ( °C ) vs Humidity ( % RH )":cluster{dbl[], dbl[]}[])
            n2142 = Build Array "Build Array"(w2289, w2412, w2410, w2411) -> (→"Air Temperature  ( °C )":cluster{dbl[], dbl[]}[])
            n2143 = Build Array "Build Array"(w2262, w2335, w2334, w2333) -> (→"Humidity ( %RH )":cluster{dbl[], dbl[]}[])
            n2144 = Build Array "Build Array"(w2290, w2421, w2420, w2419) -> (→"Coefficient Of Friction":cluster{dbl[], dbl[]}[])
            n2145 = Build Array "Build Array"(w2285, w2359, w2358, w2357) -> (→"Sample Temperature ( °C )":cluster{dbl[], dbl[]}[])
            n2146 = Build Array "Build Array"(w2263, w2403, w2405, w2404) -> (→"XY Graph 13":cluster{dbl[], dbl[]}[])
            n2147 = Bundle "Bundle"(w2271, w2294) -> (w2316:cluster{dbl[], dbl[]})  [unwired: 1 in]
            n2148 = Bundle "Bundle"(w2267, w2292) -> (w2314:cluster{dbl[], dbl[]})  [unwired: 1 in]
            n2149 = Bundle "Bundle"(w2269, w2293) -> (w2315:cluster{dbl[], dbl[]})  [unwired: 1 in]
            n2150 = Bundle "Bundle"(w2265, w2291) -> (w2313:cluster{dbl[], dbl[]})  [unwired: 1 in]
            n2151 = Build Array "Build Array"(w2316, w2315, w2314, w2313) -> (→"Stroke ( mm )":cluster{dbl[], dbl[]}[])
            n2152 = local write "XY Graph 16"(w2288) -> ()
          }
          frame #2 {
          }
          frame #3 {
            n2153 = local write "Numeric 8"(0 ("Numeric 8")) -> ()
            n2154 = local write "Numeric 11"(0 ("Numeric 11")) -> ()
            n2155 = local write "Numeric 12"(0 ("Numeric 12")) -> ()
            n2156 = local write "Numeric 13"(0 ("Numeric 13")) -> ()
            n2157 = property on="OPEN" class="Bool (strict)"("Visible"=TRUE) -> ()  [unwired: 2 in, 2 out]
            n2158 = local read "String Control 2"() -> (w2588:string)
            n2159 = local read "String Control 4"() -> (w2587:string)
            n2160 = local read "String Control 6"() -> (w2586:string)
            n2161 = local read "String Control 8"() -> (w2585:string)
            n2162 = Match Pattern(string=w2588, regular expression="Samples / cycle :- ") -> (after substring=w2602:string)  [unwired: 1 in, 3 out]
            n2163 = Match Pattern(string=w2588, regular expression="Frequency :- ") -> (after substring=w2621:string)  [unwired: 1 in, 3 out]
            n2164 = Match Pattern(string=w2587, regular expression="Samples / cycle :- ") -> (after substring=w2598:string)  [unwired: 1 in, 3 out]
            n2165 = Match Pattern(string=w2587, regular expression="Frequency :- ") -> (after substring=w2616:string)  [unwired: 1 in, 3 out]
            n2166 = Match Pattern(string=w2586, regular expression="Samples / cycle :- ") -> (after substring=w2594:string)  [unwired: 1 in, 3 out]
            n2167 = Match Pattern(string=w2586, regular expression="Frequency :- ") -> (after substring=w2611:string)  [unwired: 1 in, 3 out]
            n2168 = Match Pattern(string=w2585, regular expression="Samples / cycle :- ") -> (after substring=w2590:string)  [unwired: 1 in, 3 out]